vi "Main.vi"() -> ()   [LabVIEW 2018]
uses:
  <vilib>/Utility/config.llb/Write Key (String).vi
  <vilib>/Utility/config.llb/Read Key (String).vi
  <vilib>/Analysis/NI_AALBase.lvlib
  <vilib>/Utility/config.llb/NI_LVConfig.lvlib
panel:
  in  "Laser Power Tab":enum32{"Laser Power Control"}(tab)
  in  "Power Rotate":bool
  in  "Pulses\n(/0.45deg)":u16=10
  in  "Direction":bool=TRUE
  in  "Shutter":bool
  in  "File Tab":enum32{"File Operation for 2D Images"}(tab)
  in  "Overlap?":bool
  in  "Phasor?":bool
  in  "Experiment Name (2D)":string="2D_SAMPLE_1"
  in  "Save Directory (2D)":path=path "C:/Users/Yide/Google Drive/Experiments/[2018] Nanosecond FLIM/LabView/20180315 event driven program multiplexing 3D imaging"
  in  "Current Directory (2D)?":bool=TRUE
  in  "File Name (2D)":string="W800_P200_5mW_Ax1"
  in  "4 Mix?":bool
  in  "Intensity?":bool=TRUE
  in  "1w Lifetime?":bool
  in  "DC&1w Lifetime?":bool
  in  "1w Composite?":bool
  in  "DC&1w Composite?":bool
  in  "G?":bool=TRUE
  in  "S?":bool=TRUE
  in  "Save 2D Images":bool
  in  "Time Stamp?":bool
  in  "Crop Pixels":u16=40
  in  "Global Setting Tab":enum32{"Settings", "I/O"}(tab)
  in  "Global Parameters":T1={"DC AI Min (V)"=0.0015, "DC AI Max (V)"=0.06, "Mixer AI Min (V)"=-0.3, "Mixer AI Max (V)"=0.3, "Bias AO Min (V)"=0.0, "Bias AO Max (V)"=10.0, "Scan AO Min (V)"=-10.0, "Scan AO Max (V)"=10.0, "Fast Samp Freq (Hz)"=2500000.0, "Slow Samp Freq (Hz)"=250000.0}
  in  "LaserRepRate (Hz)":dbl=80000000.0 format="%#_6f"
  in  "Mixer AI Channel(s)":tag="DAQ_6110/ai0:3"
  in  "Bias AO Channel(s)":tag="DAQ-6323/ao0:3"
  in  "Scan AO Channel(s)":tag="DAQ_6110/ao0:1"
  in  "Stage VISA COM":refnum<visa-resource-name>="COM4"
  in  "DM Resource Name":refnum<visa-resource-name>="USB0::0x1313::0x8016::M00473655::RAW"
  in  "Use Stage?":bool
  in  "Use DM?":bool
  in  "Shutter Line":tag="DAQ_6110/port0/line0"
  in  "AIStartTrigger":tag="/DAQ_6110/ai/StartTrigger"
  in  "AOStartTrigger":tag="/DAQ_6110/ao/StartTrigger"
  in  "Power Control Direction":tag="DAQ-6323/port0/line0"
  in  "Power Control Counter":tag="DAQ-6323/ctr1"
  in  "DC AI Channel(s)":tag="DAQ-6323/ai0"
  in  "Stop":bool
  in  "Stage Tab":enum32{"Stage Control"}(tab)
  in  "Report Position":bool
  in  "Set Current Z to 0":bool
  in  "X-":bool
  in  "XY0":bool
  in  "X+":bool
  in  "Y+":bool
  in  "Y-":bool
  in  "Z+":bool
  in  "Z-":bool
  out "Z (.1um)":string="-44565\r"
  out "X (um)":string="-1668"
  out "Y (um)":string="1507"
  in  "Set Current XY to 0":bool
  in  "X Goal (um)":i32
  in  "Y Goal (um)":i32
  in  "Z Goal (.1um)":i32
  in  "Go to Any XYZ":bool
  in  "Z0":bool
  in  "XY Step (um)":u32=30
  in  "Z Step (.1um)":u32=10
  out "Timeout Indicator":bool=TRUE
  out "XY Speed (%)":string="100\r"
  out "Z Speed (%)":string="100\r"
  in  "Update?":bool=TRUE
  in  "Main Tab":T2(tab)
  in  "Wavelength #4":string="920_default"
  in  "Wavelength #3":string="860_default"
  in  "Wavelength #2":string="800_default"
  in  "Wavelength #1":string="780_default"
  in  "Wavelength (nm)":string="800"
  out "[d24]#1":dbl=-0.00027599829101562496
  out "[d13]#1":dbl=-0.0002700548828125
  out "[VIFmin]":dbl=-0.00643952880859375
  out "[VIFmax]":dbl=0.008984417724609376
  in  "Offset Cali Steps":dbl=200.0
  out "Power Off Voltages":dbl[][](graph)=[[0.0019911812034871324, 0.0019902088312526056, 0.0019976320631877676, 0.001989502609684019, 0.001989542137010473, 0.0019965252980430693, 0.0019877423260723044, 0.0019898741665543072, 0.001996886314292539, 0.0019883431414370327, 0.0019902483585793945, 0.001996488405871611, 0.0019877871237096007, 0.0019916212743898466, 0.0019964805004059533, 0.0019849859538316464, 0.001993689871148261, 0.001991950668778487, 0.0019876474604889082, 0.0019969917204968146, 0.0019898293689174207, 0.00199039856242042, 0.001995613534375968, 0.001984342975985365, 0.0019894209198759207, 0.0019860795432005748, 0.0019960878622955675, 0.001988264086784233, 0.0019909598504578175, 0.0019944119036476374, 0.001985726432416283, 0.0019903985624205047, 0.001992880878530776, 0.0019853838622526853, 0.0019917082345083503, 0.0019930284472165207, 0.0019852283881011163, 0.0019921772921172123, 0.0019914868814794543, 0.0019937425742506685, 0.001990169303926168, 0.0019869781310916817, 0.0019979403763351502, 0.0019892944324308597, 0.0019907569435147518, 0.001992912500392002, 0.001983533983367669, 0.001992071885913032, 0.0019913366776386117, 0.00198596359637612, 0.0019959402936094175, 0.0019889966599037014, 0.0019957531975967045, 0.001985412848958523, 0.001992048169517098, 0.0019875209730443547, 0.0019941562936023343, 0.001992580470848549, 0.001988000571273247, 0.001989976937603306, 0.0019929125003920706, 0.0019946727840028213, 0.001992475064644278, 0.001987539419129691, 0.001996132659932169, 0.001990980931699173, 0.001999871945027298, 0.001992717498913392, 0.0019950390705623603, 0.0019946885949334923, 0.0019868094811652534, 0.0019935950055645804, 0.001993905953867071, 0.001988158680580005, 0.0019958954959723462, 0.0019917872891615576, 0.001990327413232226, 0.0019988863970182634, 0.001989062538781203, 0.0019924882404199333, 0.001998491123752251, 0.001989112606728288, 0.00199077011929044, 0.0019972815875585466, 0.0019862692743681945, 0.001991971750019027, 0.0019946859597784043, 0.001994024535846976, 0.0019884116554699624, 0.001996406716063412, 0.0019900902492729507, 0.001989088890332149, 0.0019964646894756006, 0.001991154851935998, 0.0019884986155882566, 0.0019963250262547403, 0.001989892612640009, 0.001987310160635245, 0.001995429073518625, 0.0019907569435148316], [-0.000780029296875, -0.000785849609375, -0.000784853515625, -0.00077974609375, -0.000784716796875, -0.000781845703125, -0.000778427734375, -0.0007805859375, -0.00078244140625, -0.00079072265625, -0.000786513671875, -0.000782119140625, -0.00078134765625, -0.00078166015625, -0.000782021484375, -0.00078, -0.000782958984375, -0.000782236328125, -0.000784921875, -0.000779189453125, -0.000781240234375, -0.000781123046875, -0.0007850390625, -0.0007797265625, -0.000781376953125, -0.000785947265625, -0.000786044921875, -0.00078123046875, -0.000786796875, -0.000780068359375, -0.00078330078125, -0.0007794140625, -0.0007826171875, -0.000782041015625, -0.000785029296875, -0.000778994140625, -0.000782216796875, -0.000782333984375, -0.00077810546875, -0.000780859375, -0.000775361328125, -0.000779716796875, -0.00078251953125, -0.00078333984375, -0.00077982421875, -0.000783876953125, -0.000784658203125, -0.000783046875, -0.000786318359375, -0.000780224609375, -0.0007908203125, -0.000779169921875, -0.000781484375, -0.000784423828125, -0.000784970703125, -0.0007749609375, -0.000784765625, -0.0007823828125, -0.000785, -0.000778544921875, -0.000786865234375, -0.000784248046875, -0.00077919921875, -0.000780107421875, -0.000784833984375, -0.000776689453125, -0.000783837890625, -0.000791083984375, -0.000780732421875, -0.00078015625, -0.000789560546875, -0.0007856640625, -0.000782998046875, -0.0007909765625, -0.0007870703125, -0.000784462890625, -0.000792294921875, -0.00078140625, -0.000783408203125, -0.00078900390625, -0.000791640625, -0.00078412109375, -0.0007849609375, -0.00077884765625, -0.00077947265625, -0.000785859375, -0.000786572265625, -0.0007895703125, -0.000787041015625, -0.000784873046875, -0.000788974609375, -0.00079103515625, -0.00078923828125, -0.000784736328125, -0.00078291015625, -0.00078708984375, -0.00078943359375, -0.00078662109375, -0.000792861328125, -0.000789296875], [-0.000335673828125, -0.00034333984375, -0.00034349609375, -0.00034013671875, -0.00033658203125, -0.000334326171875, -0.000336240234375, -0.00033765625, -0.00033697265625, -0.000335712890625, -0.00033833984375, -0.000332509765625, -0.000334375, -0.000326171875, -0.000337841796875, -0.0003422265625, -0.000350634765625, -0.00033880859375, -0.000343271484375, -0.00033705078125, -0.000335634765625, -0.00033783203125, -0.0003369921875, -0.000341923828125, -0.000327080078125, -0.000332646484375, -0.000334150390625, -0.0003337109375, -0.000345732421875, -0.000341181640625, -0.000348154296875, -0.000341923828125, -0.000339677734375, -0.000340283203125, -0.00034009765625, -0.000337763671875, -0.000337578125, -0.000336474609375, -0.000333564453125, -0.00032603515625, -0.00032876953125, -0.000347666015625, -0.00034099609375, -0.0003371484375, -0.000341357421875, -0.00033509765625, -0.000343896484375, -0.000332802734375, -0.000336357421875, -0.0003353125, -0.000335244140625, -0.00033578125, -0.000331552734375, -0.0003305859375, -0.000340419921875, -0.000345419921875, -0.0003437890625, -0.000336669921875, -0.000334638671875, -0.0003310546875, -0.000333173828125, -0.000340888671875, -0.000333759765625, -0.00032828125, -0.00033412109375, -0.0003459765625, -0.00034267578125, -0.000337822265625, -0.000340673828125, -0.000339013671875, -0.00034138671875, -0.00034056640625, -0.000340185546875, -0.000335107421875, -0.000337041015625, -0.00032955078125, -0.000334638671875, -0.000328193359375, -0.000343291015625, -0.00034142578125, -0.0003435546875, -0.0003431640625, -0.0003390625, -0.0003366015625, -0.000342431640625, -0.000340322265625, -0.000333271484375, -0.00032931640625, -0.000326796875, -0.000330078125, -0.000336064453125, -0.00034599609375, -0.000336640625, -0.00034908203125, -0.000337626953125, -0.000337880859375, -0.000336240234375, -0.0003367578125, -0.000333916015625, -0.000338994140625]]
  in  "[O_B]":dbl=0.0019611298946414523
  out "[O_B]#4":dbl=0.0019817224986922125
  out "[O_B]#3":dbl=0.0019770983153341026
  out "[O_B]#2":dbl=0.0019732996865433994
  out "[M/B]#4":dbl=11.957710379168162
  out "Calibrated Bias #4":dbl[](array[numeric])=[4.030240894527995, 5.331277365972248, 7.017893239286359, 2.1441192668577616] caption="Calibrated Bias (V)"
  out "[M/B]#3":dbl=6.9445752723835525
  out "Calibrated Bias #3":dbl[](array[numeric])=[4.133266170338223, 5.459927871661395, 7.215275600866896, 2.32335998053599] caption="Calibrated Bias (V)"
  out "[M/B]#2":dbl=6.651018084174256
  out "Calibrated Bias #2":dbl[](array[numeric])=[4.266512052668534, 5.619139583144605, 7.33914581010989, 2.4564183229239265] caption="Calibrated Bias (V)"
  in  "Load #4":bool
  in  "Save #4":bool
  in  "Load #3":bool
  in  "Save #3":bool
  in  "Load #2":bool
  in  "Save #2":bool
  out "Expected Time (s)":dbl=10.0
  in  "Calibration Parameters":T3={"Target Lifetime (s)"=2.3e-09, "Integration Time (s)"=0.01, "Calibration Steps"=1000.0}
  in  "Calibrate":bool
  out "Actual Time (s)":dbl=15.825
  out "Calibrate Progress":u8(slide)=100 caption="Progress (%)" scale=0.0..100.0
  out "Calibration AI  Signals (Integrated)":dbl[][](graph)=[[-0.0025954345703125], [-0.002719150390625], [-0.002092578125], [-0.002607724609375]]
  in  "Calibrated Bias (V)":dbl[](array[numeric])=[3.4515014635363475, 4.932036093848717, -1.993, 1.1468780774213565]
  out "Mixer Phases":cluster{"X":dbl[], "Y":dbl[]}[](graph)
  in  "Save Calibration Info":bool
  in  "[M/B]":dbl=13.06780937640502
  out "Calibration AI  Signals (Integrated) 2":dbl[](graph)=[0.003525109360504571]
  out "[M/B]#1":dbl=7.8776179857171815
  out "Calibrated Bias #1":dbl[](array[numeric])=[4.358008870745989, 5.66047188871341, 7.405368893950525, 2.434138560286041] caption="Calibrated Bias (V)"
  in  "Save #1":bool
  in  "Load #1":bool
  out "[O_B] #1":dbl=0.001973990228939348
  in  "PowerOffCalibration":bool
  out "[d24]#2":dbl=-0.0003672878417968749
  out "[d13]#2":dbl=-0.00038435239257812503
  out "[d24]#3":dbl=-0.000298224609375
  out "[d13]#3":dbl=-0.00022965332031249996
  out "[d24]#4":dbl=-0.00010210942382812502
  out "[d13]#4":dbl=-1.1540429687499992e-05
  out "[V_DC]":dbl=0.014297467963349433
  in  "[d24]":dbl=0.0019611298946414523
  in  "[d13]":dbl=0.0019611298946414523
  out "Normalized Variance":dbl(graph)=0.00227571952127783
  in  "Single Pixel?":bool
  in  "Calculate Pixel Width":bool
  in  "Record X2":bool
  in  "Fast Scan Frames":u32=1000
  out "Expected Frame Time (s)":dbl=0.8
  in  "Fast Scan Parameters":T4={"Pixel Dwell Time (s)"=1.2e-05, "Pixel Size"=300.0, "X Min (V)"=-7.5, "X Max (V)"=7.5, "Y Min (V)"=-7.5, "Y Max (V)"=7.5, "XY Factor (1/V)"=0.127073}
  in  "Fast Scan":bool
  out "Actual Scan Time (s)":dbl=0.826
  out "Fast Scan Progress":dbl(slide) caption="Progress (%)" scale=0.0..100.0
  out "Fast Scan Intensity Image":dbl[][](graph)
  in  "Record X1":bool
  out "X1 (px)":dbl=217.0
  out "X2 (px)":dbl=120.0
  out "dX (nm/px)":dbl=303.030303030303
  out "New XY Factor":dbl=0.12707333333333332
  out "Mean Pixel Value":dbl(graph)=0.00227571952127783
  in  "Calculate XY Factor":bool
  in  "Objective Lens":T5(ring)
  in  "Desired Pixel Width (nm)":dbl=200.0
  in  "Calculate XY Based on Objective":bool caption="Calculate XY Factor"
  in  "Stop Fast Scan":bool
  out "Expected Frame Time (s)":dbl=3.2
  in  "Measure":bool
  out "Actual Meas Time (s)":dbl=34.819
  in  "Measurement Parameters":T4={"Pixel Dwell Time (s)"=1.2e-05, "Pixel Size"=400.0, "X Min (V)"=-7.5, "X Max (V)"=7.5, "Y Min (V)"=-7.5, "Y Max (V)"=7.5, "XY Factor (1/V)"=0.127073}
  in  "Images Tab":T6(tab)
  in  "Min (%)":dbl
  in  "Max (%)":dbl=100.0
  out "V_IF (0)":dbl[][](graph)
  out "V_IF (pi)":dbl[][](graph)
  out "V_IF (0.5pi)":dbl[][](graph)
  out "V_IF (1.5pi)":dbl[][](graph)
  out "V_DC":dbl[][](graph)
  in  "Auto Scale?":bool=TRUE
  in  "Max Intensity":dbl=0.003482028663545093
  in  "Min Intensity":dbl=0.001848886980185905
  out "std_01":dbl format="%.4g"
  out "std_1":dbl format="%.4g"
  out "DC&1w Lifetime Hist":T7(graph)={"X Values"=array[1000 elements], "Histogram: h(x)"=[1, 1, 1, 1, 3, 1, 4, 1, 0, 0, 0, 1, 1, 1, 2, 1, 4, 1, 2, 2, 1, 4, 2, 2, 2, 1, 0, 0, 2, 1, 4, 1, 0, 3, 1, 0, 4, 1, 2, 1, 1, 0, 1, 2, 0, 1, 2, 2, 2, 0, 1, 4, 0, 1, 1, 2, 0, 0, 1, 1, 1, 0, 3, 2, 0, 1, 3, 1, 4, 2, 2, 2, 1, 0, 2, 2, 2, 1, 2, 1, 4, 0, 2, 1, 3, 1, 1, 0, 1, 1, 0, 4, 3, 2, 2, 2, 2, 2, 0, 0, 0, 2, 2, 2, 1, 1, 2, 3, 2, 0, 1, 2, 2, 2, 2, 2, 0, 1, 0, 0, 3, 4, 3, 2, 0, 1, 0, 0, 1, 1, 3, 2, 1, 2, 3, 2, 2, 0, 1, 3, 1, 1, 3, 2, 1, 2, 3, 2, 0, 0, 2, 4, 2, 4, 0, 2, 1, 1, 2, 0, 1, 1, 1, 1, 0, 2, 1, 3, 0, 1, 1, 5, 7, 4, 3, 2, 2, 3, 1, 3, 2, 6, 3, 4, 1, 3, 0, 0, 2, 4, 3, 2, 2, 3, 3, 3, 5, 6, 7, 3, 2, 0, 1, 4, 8, 4, 0, 5, 4, 4, 0, 3, 4, 1, 3, 4, 4, 3, 8, 3, 3, 6, 4, 3, 6, 3, 3, 5, 2, 5, 3, 3, 4, 3, 2, 5, 3, 4, 5, 0, 7, 3, 6, 4, 7, 4, 8, 6, 5, 5, 3, 4, 6, 4, 3, 4, 4, 4, 6, 4, 5, 12, 2, 7, 4, 3, 7, 4, 5, 8, 3, 4, 2, 5, 9, 2, 10, 8, 12, 3, 3, 7, 10, 6, 10, 8, 3, 5, 7, 7, 8, 9, 10, 10, 5, 13, 13, 11, 9, 13, 15, 4, 6, 8, 9, 8, 6, 9, 21, 15, 7, 13, 6, 15, 11, 14, 12, 13, 20, 19, 14, 22, 26, 12, 16, 24, 21, 22, 30, 26, 24, 14, 26, 24, 27, 27, 44, 35, 38, 34, 55, 29, 51, 48, 56, 54, 69, 53, 55, 71, 65, 80, 84, 93, 81, 99, 79, 117, 119, 119, 123, 122, 141, 142, 152, 152, 148, 175, 155, 185, 194, 208, 210, 222, 222, 259, 265, 257, 233, 318, 276, 277, 318, 324, 340, 340, 344, 393, 389, 409, 460, 422, 408, 446, 440, 423, 456, 490, 475, 501, 479, 495, 500, 509, 508, 530, 503, 545, 563, 520, 555, 533, 589, 577, 567, 618, 585, 600, 588, 579, 617, 548, 599, 584, 577, 632, 597, 671, 623, 646, 602, 605, 617, 625, 604, 688, 638, 618, 639, 679, 632, 659, 673, 620, 660, 682, 623, 642, 684, 629, 649, 721, 639, 691, 639, 651, 645, 652, 637, 643, 673, 654, 650, 662, 651, 669, 641, 644, 619, 583, 638, 648, 622, 627, 627, 638, 647, 642, 574, 618, 588, 607, 569, 639, 593, 586, 606, 576, 559, 600, 580, 563, 584, 581, 560, 521, 565, 497, 544, 550, 542, 490, 534, 547, 503, 511, 498, 465, 480, 504, 468, 472, 484, 498, 528, 451, 513, 468, 506, 451, 447, 428, 454, 471, 453, 452, 451, 410, 448, 437, 439, 405, 411, 411, 398, 416, 413, 400, 397, 368, 367, 365, 371, 379, 363, 352, 373, 342, 365, 359, 383, 332, 369, 338, 356, 337, 341, 327, 306, 323, 324, 327, 281, 290, 310, 288, 282, 299, 288, 279, 281, 290, 247, 310, 263, 278, 292, 264, 293, 241, 244, 245, 277, 257, 254, 272, 267, 238, 273, 228, 232, 261, 219, 237, 240, 222, 216, 250, 223, 227, 241, 192, 221, 222, 220, 210, 233, 218, 182, 194, 190, 204, 228, 188, 173, 214, 197, 174, 187, 177, 204, 213, 187, 190, 191, 187, 204, 162, 179, 169, 177, 183, 161, 155, 168, 144, 177, 167, 169, 172, 163, 189, 157, 159, 138, 166, 176, 145, 160, 142, 153, 133, 170, 129, 144, 122, 131, 150, 126, 129, 145, 127, 141, 103, 127, 124, 122, 128, 119, 127, 114, 113, 115, 108, 132, 117, 122, 121, 118, 94, 123, 124, 112, 101, 124, 104, 90, 107, 111, 106, 113, 104, 105, 102, 98, 89, 99, 109, 109, 95, 97, 87, 106, 81, 109, 108, 107, 102, 89, 86, 81, 89, 88, 84, 83, 92, 90, 85, 90, 86, 97, 92, 73, 75, 87, 76, 73, 89, 80, 73, 78, 75, 59, 80, 74, 63, 86, 87, 71, 77, 66, 73, 72, 78, 85, 70, 81, 84, 70, 72, 81, 65, 71, 82, 57, 70, 65, 69, 60, 77, 71, 70, 71, 88, 69, 60, 71, 55, 66, 71, 71, 54, 59, 62, 61, 64, 65, 58, 63, 66, 64, 52, 64, 70, 56, 70, 72, 52, 51, 60, 66, 59, 59, 44, 54, 53, 49, 61, 47, 47, 35, 60, 51, 52, 48, 49, 54, 49, 50, 48, 40, 48, 47, 55, 55, 43, 41, 54, 36, 46, 51, 46, 39, 51, 42, 53, 50, 55, 41, 46, 59, 42, 44, 48, 42, 43, 45, 48, 27, 51, 40, 46, 45, 48, 46, 46, 43, 47, 48, 46, 30, 33, 43, 34, 48, 50, 39, 33, 44, 51, 26, 49, 46, 41, 37, 41, 42, 42, 47, 43, 39, 39, 39, 40, 35, 36, 41, 33, 35, 31, 43, 37, 36, 41, 26, 35, 35, 23, 36, 29, 38, 35, 38, 28, 33, 43, 38, 25, 34, 34, 40, 38, 33, 31, 32, 27, 35, 36, 28, 33, 36, 35, 37, 34, 30, 34, 25, 27, 28, 26, 35, 30, 37, 30, 28, 23, 30, 36, 17, 28, 28, 23, 25, 26, 36, 37, 33, 23, 31, 31, 22, 35, 25, 27, 24, 32, 25, 27, 25, 27, 24, 35, 26, 33, 20, 30, 15, 23, 29, 23, 30, 33, 32, 22, 20, 35, 27, 22, 28, 21, 22, 18, 20, 23, 22, 16, 22, 18, 34, 20, 26, 28, 25, 10, 20, 27, 26, 30, 19, 18, 25, 21, 21, 24, 28, 22, 23, 23, 22, 22]}
  out "DC&1w Lifetime (s)":dbl[][](graph)
  in  "Bins":i32=1000
  in  "Lifetime Selection":enum32{"1w Lifetime", "DC&1w Lifetime"}(radio) caption="Radio Buttons"
  out "Composite Image":picture caption="HSV to RGB Picture"
  in  "Max Lifetime (s)":dbl=4e-09
  in  "Min Lifetime (s)":dbl=1e-09
  out "Lifetime Color Ramp":i32[][](graph) caption="Vertical Color Ramp"
  out "1w Lifetime (s)":dbl[][](graph)
  out "1w Lifetime Hist":T7(graph)={"X Values"=array[1000 elements], "Histogram: h(x)"=[13, 27, 13, 19, 32, 22, 15, 16, 16, 16, 27, 21, 25, 18, 27, 21, 28, 22, 34, 24, 28, 18, 33, 20, 27, 26, 27, 35, 17, 17, 25, 33, 24, 20, 14, 23, 24, 30, 31, 35, 36, 32, 29, 19, 23, 24, 22, 23, 22, 25, 31, 29, 24, 36, 32, 25, 22, 34, 30, 39, 30, 33, 34, 23, 23, 32, 31, 32, 25, 28, 53, 27, 40, 37, 36, 42, 35, 26, 32, 36, 44, 53, 29, 28, 45, 37, 50, 37, 35, 35, 35, 33, 44, 50, 40, 42, 41, 41, 36, 41, 40, 37, 51, 51, 55, 61, 32, 37, 66, 54, 44, 46, 41, 42, 51, 52, 53, 40, 46, 50, 53, 49, 52, 57, 46, 51, 57, 60, 51, 60, 48, 46, 54, 62, 47, 56, 58, 59, 47, 40, 62, 54, 61, 68, 62, 78, 68, 74, 84, 66, 70, 64, 68, 71, 77, 78, 62, 64, 61, 95, 87, 79, 71, 85, 76, 62, 69, 69, 83, 67, 73, 87, 71, 86, 91, 87, 101, 82, 83, 90, 101, 107, 84, 90, 90, 94, 114, 100, 99, 107, 100, 88, 109, 93, 104, 106, 126, 128, 120, 129, 117, 112, 130, 126, 140, 127, 130, 151, 131, 124, 138, 138, 186, 151, 149, 152, 175, 152, 154, 164, 162, 149, 161, 164, 175, 156, 185, 170, 169, 199, 191, 215, 214, 184, 187, 201, 207, 206, 219, 264, 235, 237, 242, 253, 258, 273, 287, 286, 268, 284, 278, 291, 293, 277, 312, 311, 361, 330, 342, 291, 363, 351, 342, 335, 346, 379, 400, 399, 395, 408, 397, 387, 434, 500, 425, 431, 481, 473, 506, 504, 459, 511, 518, 510, 540, 551, 511, 515, 590, 529, 609, 631, 587, 578, 607, 626, 625, 622, 643, 660, 636, 696, 623, 691, 708, 679, 754, 723, 723, 764, 733, 725, 784, 780, 795, 787, 842, 804, 837, 826, 826, 848, 884, 878, 840, 911, 890, 886, 850, 834, 905, 891, 923, 968, 928, 894, 881, 931, 847, 921, 934, 903, 895, 935, 938, 876, 851, 857, 909, 974, 892, 877, 827, 888, 909, 861, 842, 857, 830, 861, 807, 880, 846, 904, 785, 861, 780, 760, 783, 728, 761, 730, 714, 721, 701, 680, 677, 688, 658, 657, 636, 642, 588, 614, 609, 592, 600, 555, 603, 556, 536, 537, 538, 484, 525, 533, 483, 456, 476, 470, 432, 454, 435, 429, 477, 417, 404, 381, 368, 403, 398, 402, 378, 354, 367, 336, 339, 339, 327, 333, 263, 304, 296, 299, 294, 316, 247, 276, 251, 233, 267, 247, 239, 245, 217, 260, 230, 242, 212, 187, 223, 181, 208, 204, 189, 207, 196, 174, 191, 182, 167, 168, 178, 146, 170, 174, 154, 160, 161, 153, 156, 136, 131, 143, 152, 147, 120, 138, 124, 107, 120, 127, 110, 100, 93, 107, 94, 115, 99, 110, 88, 92, 98, 90, 90, 100, 101, 91, 77, 97, 84, 99, 87, 74, 73, 66, 84, 72, 86, 88, 63, 73, 85, 76, 74, 66, 67, 68, 69, 65, 63, 69, 49, 62, 54, 63, 52, 51, 49, 54, 60, 54, 50, 45, 55, 52, 60, 67, 53, 52, 47, 56, 48, 48, 36, 41, 44, 56, 51, 37, 39, 45, 36, 39, 41, 43, 45, 51, 47, 41, 36, 33, 36, 35, 29, 34, 50, 40, 28, 33, 34, 31, 22, 30, 29, 30, 42, 25, 30, 33, 39, 23, 33, 29, 33, 26, 32, 33, 29, 29, 32, 36, 29, 30, 34, 39, 29, 29, 28, 29, 29, 27, 30, 33, 23, 22, 31, 28, 28, 21, 22, 32, 21, 26, 22, 15, 29, 24, 16, 31, 27, 22, 26, 20, 32, 30, 21, 22, 26, 12, 26, 23, 23, 18, 17, 24, 22, 28, 20, 25, 28, 23, 17, 17, 20, 40, 24, 19, 29, 24, 19, 20, 19, 22, 19, 26, 16, 25, 22, 15, 19, 20, 20, 20, 16, 19, 24, 20, 27, 11, 26, 19, 14, 22, 26, 20, 15, 16, 28, 19, 24, 20, 20, 13, 17, 32, 22, 22, 19, 22, 23, 22, 21, 17, 19, 9, 17, 10, 19, 21, 12, 18, 16, 12, 20, 16, 18, 15, 15, 12, 20, 13, 25, 17, 17, 20, 18, 11, 15, 20, 18, 18, 12, 19, 25, 16, 15, 16, 20, 16, 12, 17, 18, 19, 16, 8, 16, 16, 15, 15, 6, 18, 13, 14, 18, 17, 10, 21, 18, 13, 13, 12, 12, 18, 13, 22, 16, 19, 14, 23, 10, 14, 15, 10, 18, 7, 17, 9, 17, 14, 17, 13, 11, 6, 19, 15, 14, 11, 10, 10, 11, 9, 10, 11, 10, 23, 13, 15, 9, 12, 11, 10, 15, 15, 13, 12, 12, 13, 7, 10, 9, 10, 15, 4, 13, 8, 12, 10, 9, 7, 12, 11, 13, 10, 7, 10, 9, 11, 13, 9, 7, 11, 13, 11, 10, 12, 14, 6, 12, 10, 7, 13, 8, 8, 12, 8, 12, 15, 9, 15, 6, 14, 9, 12, 6, 9, 9, 10, 10, 5, 12, 6, 10, 11, 12, 7, 7, 11, 10, 18, 8, 5, 4, 11, 10, 9, 6, 5, 10, 10, 5, 6, 9, 8, 11, 5, 11, 10, 5, 5, 8, 14, 7, 5, 12, 7, 9, 7, 8, 2, 8, 11, 9, 4, 10, 7, 6, 7, 6, 6, 7, 3, 9, 4, 10, 11, 4, 5, 10, 6, 10, 3, 8, 8, 9, 8, 7, 9, 3, 6, 7, 6, 3, 11, 9, 7, 5, 8, 6, 9, 10, 9, 8, 5, 8, 9, 4, 5, 7, 2, 8, 3, 4, 4, 6, 7, 7, 4, 4, 5, 8, 4, 4, 7, 5, 8, 7, 6, 6, 7, 4, 5, 7, 1, 5, 8, 5, 9, 3, 4, 6, 6, 8, 9, 4, 4, 5, 7, 7, 8, 4, 3, 4, 7, 9, 7, 4, 5, 6, 3, 7, 5, 7, 2, 3, 5, 3, 5, 2, 2, 3, 3, 11, 0, 5, 4, 0, 9, 4, 7]}
  out "u_1w":dbl format="%.4g"
  out "u_01":dbl format="%.4g"
  in  "Update Phasor":bool
  in  "S_min":dbl=-0.1
  in  "S_max":dbl=1.1
  in  "G_min":dbl=-0.1
  in  "G_max":dbl=1.1
  in  "ROI4?":bool
  in  "ROI3?":bool
  in  "ROI2?":bool
  in  "Color4":u32(colorbox)=16860
  out "Center4":cluster{dbl, dbl}={0.3861111111111111, 0.4194444444444444}
  in  "Color3":u32(colorbox)=9567230
  out "Center3":cluster{dbl, dbl}={0.4777777777777778, 0.4277777777777777}
  in  "Color2":u32(colorbox)=6618880
  out "Center2":cluster{dbl, dbl}={0.4444444444444445, 0.4916666666666667}
  in  "ROI Select":enum16{"None", "ROI1", "ROI2", "ROI3", "ROI4"}(ring)
  in  "Color1":u32(colorbox)=16711680
  in  "Phasor Grids":i32=400
  out "G Data":dbl[][](array[numeric])
  out "S Data":dbl[][](array[numeric])
  out "G":dbl=-0.16111111111111112
  out "S":dbl=0.5888888888888888
  out "[tau]":dbl=-7.271734468853837e-09
  out "Phasor Plot":dbl[][](graph)
  out "Center1":cluster{dbl, dbl}={0.45, 0.4194444444444444}
  out "Radius1":dbl=0.03621779114001471
  out "Radius2":dbl=0.03621779114001474
  out "Radius3":dbl=0.025609845714702418
  out "Radius4":dbl=0.0496903994999953
  out "ROI Drawing":bool
  in  "ROI1?":bool
  in  "PicSize":u32=360
  out "Image with Phasors":picture caption="HSV to RGB Picture"
  in  "Phasor Colormap":T8(ring)=enum."rainbow"
  in  "Refresh Overlap":bool
  in  "Phasor\nOverlap?":bool
  out "ROI Cluster":T9
  in  "Calculate Lifetimes and Phasors During Image Acquisition?":bool=TRUE
  out "3D S":dbl[][][](array[numeric])
  out "3D G":dbl[][][](array[numeric])
  in  "Current Directory (3D)?":bool=TRUE
  in  "Save Directory (3D)":path=path "C:/Users/Yide/Google Drive/Experiments"
  in  "File Name (3D)":string="W800_P200_5mW_Ax1_dz05um"
  in  "Experiment Name (3D)":string="3D_SAMPLE_1"
  in  "Save 3D Stacks":bool
  in  "Slice Slider":i32(c297)=34
  in  "Stop Stack Measure":bool
  out "Stack Progress":dbl(slide)=100.0 caption="Progress (%)" scale=0.0..100.0
  out "Initial Z Pos (.1um)":i32=3193
  out "Current Slice":i32
  in  "Z Slice Number":i32=30
  in  "Z Slice Size (.1um)":i32=5
  in  "Z-Stack Measure":bool
  out "Slice of 3D Stack":picture caption="HSV to RGB Picture"
  out "Slice Display":string="Slice #: 35/200"
  out "Number of Slices":i32=200
  out "3D Intensity":dbl[][][](array[numeric])
  in  "3D Stack to Show":T10(ring)
  out "Time Stamp (s)":dbl=30.0
  out "Current 3D Time-Lapse Meas":i32
  in  "2D Time-Lapse Measure":bool
  in  "3D Time-Lapse Measure":bool
  out "2D Time-Lapse Progress":dbl(slide)=100.0 caption="Progress (%)" scale=0.0..100.0
  in  "Total 2D Time-Lapse Meas":i32=5
  in  "2D Time-Lapse Interval (s)":dbl=30.0
  out "3D Time-Lapse Progress":dbl(slide)=100.0 caption="Progress (%)" scale=0.0..100.0
  in  "Total 3D Time-Lapse Meas":i32=5
  in  "3D Time-Lapse Interval (s)":dbl=30.0
  out "Current 2D Time-Lapse Meas":i32
  in  "Stop 2D Time-Lapse":bool
  in  "Stop 3D Time-Lapse":bool
  out "Time Elapse (s)":dbl
  out "Angle GSOS":dbl[][](array[numeric])
  out "Angle q1,2":dbl[][](array[numeric])
  in  "qGSmin":dbl=0.02
  in  "qGSmax":dbl=0.02
  in  "q1,2min":dbl=0.02
  in  "q1,2max":dbl=0.02
  in  "q1,1min":dbl=0.02
  in  "Two-Step GSOS":bool
  in  "P2 Power (au)":dbl=6.0
  in  "Load P2":bool
  out "DC,SOS":dbl[][](graph)
  out "Mag GSOS":dbl[][](graph)
  out "DC,2":dbl[][](graph)
  out "Mag q1,2":dbl[][](graph)
  out "Mag q1,1":dbl[][](graph)
  out "DC,1":dbl[][](graph)
  in  "Load P1":bool
  in  "P1 Power (au)":dbl=5.0
  in  "q1,1max":dbl=0.02
  out "Angle q1,1":dbl[][](array[numeric])
  out "Composite GSOS":picture caption="HSV to RGB Picture"
  out "Lifetime GSOS":dbl[][](graph)
  out "Composite q1,2":picture caption="HSV to RGB Picture"
  out "Lifetime q1,2":dbl[][](graph)
  in  "Export GSOS Images":bool
  out "Lifetime q1,1":dbl[][](graph)
  out "Composite q1,1":picture caption="HSV to RGB Picture"
  in  "tau_max (s)":dbl=3e-09
  in  "tau_min (s)":dbl=1e-09
  in  "Custom Mag?":bool
  in  "# of Frames to Average":u32=1
  out "Meas Progress":dbl(slide) caption="Progress (%)" scale=0.0..100.0
  in  "Stop Measure":bool
  in  "Single Pixel Measure?":bool
  in  "Refresh":bool
  out "Metric Calibration":dbl[][](graph)
  in  "Z Cali Step":dbl=0.01
  in  "Export Z Calibration":bool
  out "Initial Metric":dbl
  out "Initial Zernike":dbl[](array[numeric])
  in  "Bias Amplitude":dbl=0.25
  in  "Load Zernike":bool
  in  "Save Zernike":bool
  in  "Quadratic Search":bool
  in  "Optimization Metric":T11(ring)
  in  "Apply Zernike":bool
  out "Z Direction":bool
  out "Current Z Idx":i32
  in  "Zernike Array":dbl[](array[slide])=[0.0, 0.0, 0.0, 0.0, 0.0, 0.0, 0.0, 0.0, 0.0, 0.0, 0.0, 0.0] min=-1.0 max=1.0 step=0.05 scale=-1.0..1.0 scale format="%#.4g"
  in  "Zernike Enable":bool[](array[boolean])=[TRUE, TRUE, TRUE, TRUE, TRUE, TRUE, TRUE, TRUE, TRUE, TRUE, TRUE, TRUE]
  in  "SPGD":bool
  in  "Learning Rate":dbl=-0.01
  in  "Relax DM":bool
  in  "Simple Max Search":bool
  out "Current Iteration":sgl
  in  "Total Iteration":u32=40
  in  "Reset Zernike":bool
  out "Last Metric":dbl
  out "Sigma":dbl[](array[numeric])
  out "Last Zernike":dbl[](array[numeric])
  in  "Stop AO Algorithm":bool
  in  "Step Size":dbl=0.05
  out "Metric Value":dbl(graph)=0.00227571952127783
  out "Optimal Zernike":dbl[](array[numeric])
  out "Quadratic Calc":bool
  out "Optimal Z Idx":i32
  in  "Note":string="Cou6_200x200_5mW_1580nm_step0.01"
  # "Instant FLIM @ Univeristy of Notre Dame  by  Yide Zhang"
  # "80MHz for\nTi:sapphire laser"
  # "Card 1 (Mixer + Scan)"
  # "Card 2 (DC + Bias)"
  # "Optional"
  # "Up"
  # "Right"
  # "Left"
  # "Down"
  # "Standard Lifetimes (s):\nCoumarin 6 MeOH - 2.3E-9\nCoumarin 6 EtOH - 2.41E-9\nFluorescein NaOH - 4.0E-9\nRhodamine B H2O - 1.7E-9"
  # "V_IF (0 or -2pi)"
  # "(Shutter On)"